vi "SaccadeAnalyser - Main.vi"(8 "error in (no error)":errorcluster, 11 "Data IN":T3={"Impulse Positions"=[{"Start"=5471, "End"=5813, "Impulse Plane"=enum."Yaw", "Impulse Direction +ve?"=FALSE, "Time offset"=0, "Amplitude offset"=0.0}, {"Start"=6974, "End"=7325, "Impulse Plane"=enum."Yaw", "Impulse Direction +ve?"=TRUE, "Time offset"=0, "Amplitude offset"=0.0}, {"Start"=7641, "End"=7980, "Impulse Plane"=enum."Yaw", "Impulse Direction +ve?"=FALSE, "Time offset"=0, "Amplitude offset"=0.0}, {"Start"=9060, "End"=9400, "Impulse Plane"=enum."Yaw", "Impulse Direction +ve?"=FALSE, "Time offset"=0, "Amplitude offset"=0.0}, {"Start"=9938, "End"=10282, "Impulse Plane"=enum."Yaw", "Impulse Direction +ve?"=FALSE, "Time offset"=0, "Amplitude offset"=0.0}, {"Start"=10800, "End"=11142, "Impulse Plane"=enum."Yaw", "Impulse Direction +ve?"=FALSE, "Time offset"=0, "Amplitude offset"=0.0}, {"Start"=11602, "End"=11942, "Impulse Plane"=enum."Yaw", "Impulse Direction +ve?"=TRUE, "Time offset"=0, "Amplitude offset"=0.0}, {"Start"=12449, "End"=12790, "Impulse Plane"=enum."Yaw", "Impulse Direction +ve?"=TRUE, "Time offset"=0, "Amplitude offset"=0.0}, {"Start"=13310, "End"=13653, "Impulse Plane"=enum."Yaw", "Impulse Direction +ve?"=TRUE, "Time offset"=0, "Amplitude offset"=0.0}, {"Start"=14191, "End"=14535, "Impulse Plane"=enum."Yaw", "Impulse Direction +ve?"=TRUE, "Time offset"=0, "Amplitude offset"=0.0}, {"Start"=15040, "End"=15380, "Impulse Plane"=enum."Yaw", "Impulse Direction +ve?"=FALSE, "Time offset"=0, "Amplitude offset"=0.0}, {"Start"=16780, "End"=17124, "Impulse Plane"=enum."Yaw", "Impulse Direction +ve?"=TRUE, "Time offset"=0, "Amplitude offset"=0.0}, {"Start"=17572, "End"=17913, "Impulse Plane"=enum."Yaw", "Impulse Direction +ve?"=FALSE, "Time offset"=0, "Amplitude offset"=0.0}, {"Start"=18369, "End"=18713, "Impulse Plane"=enum."Yaw", "Impulse Direction +ve?"=FALSE, "Time offset"=0, "Amplitude offset"=0.0}, {"Start"=19174, "End"=19519, "Impulse Plane"=enum."Yaw", "Impulse Direction +ve?"=FALSE, "Time offset"=0, "Amplitude offset"=0.0}, {"Start"=19928, "End"=20270, "Impulse Plane"=enum."Yaw", "Impulse Direction +ve?"=TRUE, "Time offset"=0, "Amplitude offset"=0.0}, {"Start"=20762, "End"=21121, "Impulse Plane"=enum."Yaw", "Impulse Direction +ve?"=FALSE, "Time offset"=0, "Amplitude offset"=0.0}, {"Start"=21554, "End"=21888, "Impulse Plane"=enum."Yaw", "Impulse Direction +ve?"=FALSE, "Time offset"=0, "Amplitude offset"=0.0}, {"Start"=22293, "End"=22639, "Impulse Plane"=enum."Yaw", "Impulse Direction +ve?"=TRUE, "Time offset"=0, "Amplitude offset"=0.0}, {"Start"=23109, "End"=23464, "Impulse Plane"=enum."Yaw", "Impulse Direction +ve?"=TRUE, "Time offset"=0, "Amplitude offset"=0.0}, {"Start"=23868, "End"=24215, "Impulse Plane"=enum."Yaw", "Impulse Direction +ve?"=TRUE, "Time offset"=0, "Amplitude offset"=0.0}, {"Start"=24643, "End"=24992, "Impulse Plane"=enum."Yaw", "Impulse Direction +ve?"=FALSE, "Time offset"=0, "Amplitude offset"=0.0}, {"Start"=25685, "End"=26023, "Impulse Plane"=enum."Yaw", "Impulse Direction +ve?"=FALSE, "Time offset"=0, "Amplitude offset"=0.0}, {"Start"=26431, "End"=26768, "Impulse Plane"=enum."Yaw", "Impulse Direction +ve?"=FALSE, "Time offset"=0, "Amplitude offset"=0.0}, {"Start"=27251, "End"=27595, "Impulse Plane"=enum."Yaw", "Impulse Direction +ve?"=FALSE, "Time offset"=0, "Amplitude offset"=0.0}, {"Start"=28832, "End"=29180, "Impulse Plane"=enum."Yaw", "Impulse Direction +ve?"=TRUE, "Time offset"=0, "Amplitude offset"=0.0}, {"Start"=31028, "End"=31383, "Impulse Plane"=enum."LARP", "Impulse Direction +ve?"=FALSE, "Time offset"=0, "Amplitude offset"=0.0}, {"Start"=32603, "End"=32936, "Impulse Plane"=enum."LARP", "Impulse Direction +ve?"=TRUE, "Time offset"=0, "Amplitude offset"=0.0}, {"Start"=33445, "End"=33779, "Impulse Plane"=enum."LARP", "Impulse Direction +ve?"=TRUE, "Time offset"=0, "Amplitude offset"=0.0}, {"Start"=34276, "End"=34629, "Impulse Plane"=enum."LARP", "Impulse Direction +ve?"=FALSE, "Time offset"=0, "Amplitude offset"=0.0}, {"Start"=35114, "End"=35460, "Impulse Plane"=enum."LARP", "Impulse Direction +ve?"=FALSE, "Time offset"=0, "Amplitude offset"=0.0}, {"Start"=35981, "End"=36324, "Impulse Plane"=enum."LARP", "Impulse Direction +ve?"=TRUE, "Time offset"=0, "Amplitude offset"=0.0}, {"Start"=36920, "End"=37249, "Impulse Plane"=enum."LARP", "Impulse Direction +ve?"=TRUE, "Time offset"=0, "Amplitude offset"=0.0}, {"Start"=37988, "End"=38322, "Impulse Plane"=enum."LARP", "Impulse Direction +ve?"=TRUE, "Time offset"=0, "Amplitude offset"=0.0}, {"Start"=38964, "End"=39324, "Impulse Plane"=enum."LARP", "Impulse Direction +ve?"=FALSE, "Time offset"=0, "Amplitude offset"=0.0}, {"Start"=39948, "End"=40284, "Impulse Plane"=enum."LARP", "Impulse Direction +ve?"=TRUE, "Time offset"=0, "Amplitude offset"=0.0}, {"Start"=40958, "End"=41293, "Impulse Plane"=enum."LARP", "Impulse Direction +ve?"=TRUE, "Time offset"=0, "Amplitude offset"=0.0}, {"Start"=41899, "End"=42229, "Impulse Plane"=enum."LARP", "Impulse Direction +ve?"=TRUE, "Time offset"=0, "Amplitude offset"=0.0}, {"Start"=42801, "End"=43154, "Impulse Plane"=enum."LARP", "Impulse Direction +ve?"=FALSE, "Time offset"=0, "Amplitude offset"=0.0}, {"Start"=43641, "End"=43980, "Impulse Plane"=enum."LARP", "Impulse Direction +ve?"=TRUE, "Time offset"=0, "Amplitude offset"=0.0}, {"Start"=44466, "End"=44821, "Impulse Plane"=enum."LARP", "Impulse Direction +ve?"=FALSE, "Time offset"=0, "Amplitude offset"=0.0}, {"Start"=45388, "End"=45722, "Impulse Plane"=enum."LARP", "Impulse Direction +ve?"=TRUE, "Time offset"=0, "Amplitude offset"=0.0}, {"Start"=46149, "End"=46510, "Impulse Plane"=enum."LARP", "Impulse Direction +ve?"=FALSE, "Time offset"=0, "Amplitude offset"=0.0}, {"Start"=47874, "End"=48206, "Impulse Plane"=enum."LARP", "Impulse Direction +ve?"=TRUE, "Time offset"=0, "Amplitude offset"=0.0}, {"Start"=50143, "End"=50479, "Impulse Plane"=enum."RALP", "Impulse Direction +ve?"=TRUE, "Time offset"=0, "Amplitude offset"=0.0}, {"Start"=50976, "End"=51310, "Impulse Plane"=enum."RALP", "Impulse Direction +ve?"=FALSE, "Time offset"=0, "Amplitude offset"=0.0}, {"Start"=51892, "End"=52226, "Impulse Plane"=enum."RALP", "Impulse Direction +ve?"=FALSE, "Time offset"=0, "Amplitude offset"=0.0}, {"Start"=52839, "End"=53171, "Impulse Plane"=enum."RALP", "Impulse Direction +ve?"=FALSE, "Time offset"=0, "Amplitude offset"=0.0}, {"Start"=53676, "End"=54012, "Impulse Plane"=enum."RALP", "Impulse Direction +ve?"=TRUE, "Time offset"=0, "Amplitude offset"=0.0}, {"Start"=54530, "End"=54877, "Impulse Plane"=enum."RALP", "Impulse Direction +ve?"=FALSE, "Time offset"=0, "Amplitude offset"=0.0}, {"Start"=55371, "End"=55711, "Impulse Plane"=enum."RALP", "Impulse Direction +ve?"=TRUE, "Time offset"=0, "Amplitude offset"=0.0}, {"Start"=56153, "End"=56482, "Impulse Plane"=enum."RALP", "Impulse Direction +ve?"=FALSE, "Time offset"=0, "Amplitude offset"=0.0}, {"Start"=57053, "End"=57390, "Impulse Plane"=enum."RALP", "Impulse Direction +ve?"=FALSE, "Time offset"=0, "Amplitude offset"=0.0}, {"Start"=57954, "End"=58292, "Impulse Plane"=enum."RALP", "Impulse Direction +ve?"=FALSE, "Time offset"=0, "Amplitude offset"=0.0}, {"Start"=58794, "End"=59130, "Impulse Plane"=enum."RALP", "Impulse Direction +ve?"=TRUE, "Time offset"=0, "Amplitude offset"=0.0}, {"Start"=59587, "End"=59931, "Impulse Plane"=enum."RALP", "Impulse Direction +ve?"=TRUE, "Time offset"=0, "Amplitude offset"=0.0}, {"Start"=60399, "End"=60744, "Impulse Plane"=enum."RALP", "Impulse Direction +ve?"=FALSE, "Time offset"=0, "Amplitude offset"=0.0}, {"Start"=61218, "End"=61559, "Impulse Plane"=enum."RALP", "Impulse Direction +ve?"=FALSE, "Time offset"=0, "Amplitude offset"=0.0}, {"Start"=62100, "End"=62442, "Impulse Plane"=enum."RALP", "Impulse Direction +ve?"=FALSE, "Time offset"=0, "Amplitude offset"=0.0}, {"Start"=62989, "End"=63322, "Impulse Plane"=enum."RALP", "Impulse Direction +ve?"=FALSE, "Time offset"=0, "Amplitude offset"=0.0}, {"Start"=63787, "End"=64136, "Impulse Plane"=enum."RALP", "Impulse Direction +ve?"=TRUE, "Time offset"=0, "Amplitude offset"=0.0}, {"Start"=64603, "End"=64953, "Impulse Plane"=enum."RALP", "Impulse Direction +ve?"=FALSE, "Time offset"=0, "Amplitude offset"=0.0}, {"Start"=65462, "End"=65795, "Impulse Plane"=enum."RALP", "Impulse Direction +ve?"=FALSE, "Time offset"=0, "Amplitude offset"=0.0}, {"Start"=66308, "End"=66645, "Impulse Plane"=enum."RALP", "Impulse Direction +ve?"=FALSE, "Time offset"=0, "Amplitude offset"=0.0}, {"Start"=67052, "End"=67402, "Impulse Plane"=enum."RALP", "Impulse Direction +ve?"=TRUE, "Time offset"=0, "Amplitude offset"=0.0}], "No. Imp"=15, "Parameter Time Series"=[{"time offset"=0.0, "Offset"=0.0, "Gain"=1.0, "inverse"=FALSE, "filter data"=FALSE, "dots"=FALSE, "interpolate"=FALSE, "List 1"=5, "Color Box"=6618880, "Boolean"=TRUE}, {"time offset"=0.0, "Offset"=0.0, "Gain"=1.0, "inverse"=FALSE, "filter data"=FALSE, "dots"=FALSE, "interpolate"=FALSE, "List 1"=6, "Color Box"=6618880, "Boolean"=FALSE}, {"time offset"=0.0, "Offset"=0.0, "Gain"=1.0, "inverse"=FALSE, "filter data"=FALSE, "dots"=FALSE, "interpolate"=FALSE, "List 1"=7, "Color Box"=6618880, "Boolean"=FALSE}, {"time offset"=0.0, "Offset"=0.0, "Gain"=1.0, "inverse"=FALSE, "filter data"=FALSE, "dots"=FALSE, "interpolate"=FALSE, "List 1"=13, "Color Box"=16777224, "Boolean"=TRUE}, {"time offset"=0.0, "Offset"=0.0, "Gain"=1.0, "inverse"=FALSE, "filter data"=FALSE, "dots"=FALSE, "interpolate"=FALSE, "List 1"=14, "Color Box"=16777224, "Boolean"=FALSE}, {"time offset"=0.0, "Offset"=0.0, "Gain"=1.0, "inverse"=FALSE, "filter data"=FALSE, "dots"=FALSE, "interpolate"=FALSE, "List 1"=15, "Color Box"=16777224, "Boolean"=FALSE}], "Parameter Impuls Series"=[{"Color"=6618880, "Visible"=TRUE, "Channel"=1, "Invert"=FALSE, "Desaccade"=FALSE, "Offset"=0.0, "Gain"=1.0}, {"Color"=6618880, "Visible"=FALSE, "Channel"=6, "Invert"=FALSE, "Desaccade"=FALSE, "Offset"=0.0, "Gain"=1.0}, {"Color"=6618880, "Visible"=FALSE, "Channel"=7, "Invert"=FALSE, "Desaccade"=FALSE, "Offset"=0.0, "Gain"=1.0}, {"Color"=16777224, "Visible"=TRUE, "Channel"=13, "Invert"=FALSE, "Desaccade"=FALSE, "Offset"=0.0, "Gain"=1.0}, {"Color"=16777224, "Visible"=FALSE, "Channel"=14, "Invert"=FALSE, "Desaccade"=FALSE, "Offset"=0.0, "Gain"=1.0}, {"Color"=16777224, "Visible"=FALSE, "Channel"=15, "Invert"=FALSE, "Desaccade"=FALSE, "Offset"=0.0, "Gain"=1.0}], "Experiment Parameters"={"Freq"=0.0, "Vel"=0, "Acc"=0, "Stimulus"="Head Impulse"}, "Autosort File"=refnum, "Data File"={"Data Channels"=array34x71049[2415666 elements], "Sample Rate"=500, "Channel List"=["Hz Position-in-Head", "Hz Velocity-in-Head", "Hy Position-in-Head", "Hy Velocity-in-Head", "Hx Position-in-Head", "Hx Velocity-in-Head", "Hl Velocity-in-Head", "Hr Velocity-in-Head", "Lx Position-in-Head", "Ly Position-in-Head", "Lz Position-in-Head", "Lx Velocity-in-Head", "Ly Velocity-in-Head", "Lz Velocity-in-Head", "Ll Velocity-in-Head", "Lr Velocity-in-Head", "Rx Position-in-Head", "Ry Position-in-Head", "Rz Position-in-Head", "Rx Velocity-in-Head", "Ry Velocity-in-Head", "Rz Velocity-in-Head", "Rl Velocity-in-Head", "Rr Velocity-in-Head", "Target on/off", "aux input 1", "aux input 2", " ", "", "", "", "Target Hor", "Target Ver", ""]}, "Experiment data path"=path "C:/Users/w.figtree/Desktop/Coils Data/3", "Image data path"=path "/Macintosh HD/Users/patrick/Studium/Diploma Thesis/Data Analysis", "LVS data path"=path "/Macintosh HD/Users/patrick/Studium/Diploma Thesis/Data Analysis", "Raw copy path"=path "/Macintosh HD/Users/patrick/Studium/Diploma Thesis/Data Analysis", "filename"="passive_lvs.lvs", "desaccading parameters"={"Tolerance"=3, "Acc Range"=7000.0, "Sample Rate"=500, "Impulse Plane 2"=enum."Yaw", "Impulse dir"=FALSE}, "Experiment Parameters 2"={"Subject"="SE Trial Short Term", "Strain"="", "Rotation plane"="", "Experimenter"=" ", "Trial"=0.0, "Time"=0.0}, "Excel"={"Excel._Application"=refnum, "Use Excel"=TRUE, "Worksheet SINE"=refnum, "Row SINE"=0, "Worksheet TRANS"=refnum, "Row TRANS"=0}, "Session Config File"=refnum, "Autosort Parameter Set"=4, "EMA Version"="EMA 2016a", "desacc "={"Threshold 1 [Acc]"=7000.0, "Threshold 2 [% of TH1]"=60, "tolerance"=3, "Search WD "=0.1, " always use TH2"=FALSE, "Range"=3.0, "Max time"=120.0, "Min time"=20.0, "Velocity Threshold"=150}, "Cycle Nr for Saccades"={"POS"=0, "NEG"=0}, "calibration name"="u_calibration_1_p00001s001_calib.mat", "Excel"=refnum} {"Parameter Time Series"."time offset" format="%.3f"; "Parameter Time Series"."Gain" format="%.1f"; "Parameter Time Series"."Offset" format="%.1f"; "Parameter Time Series"."List 1" items=["Motor-Pos", "Motor-Vel", "Lx Position-in-Head", "Ly Position-in-Head", "Lz Position-in-Head", "Lx Velocity-in-Head", "Ly Velocity-in-Head", "Lz Velocity-in-Head", "Ll Velocity-in-Head", "Lr Velocity-in-Head", "Lx Accel-in-Head", "Ly Accel-in-Head", "Lz Accel-in-Head", "Rx Position-in-Head", "Ry Position-in-Head", "Rz Position-in-Head", "Rx Velocity-in-Head", "Ry Velocity-in-Head", "Rz Velocity-in-Head", "Rl Velocity-in-Head", "Rr Velocity-in-Head", "Rx Accel-in-Head", "Ry Accel-in-Head", "Rz Accel-in-Head", "Global Trigger", "", "", ""]; "Parameter Impuls Series"."Gain" format="%.1f"; "Parameter Impuls Series"."Offset" format="%.1f"}) -> (0 "error out":errorcluster, 3 "Data OUT":T3={"Impulse Positions"=[{"Start"=5471, "End"=5813, "Impulse Plane"=enum."Yaw", "Impulse Direction +ve?"=FALSE, "Time offset"=0, "Amplitude offset"=0.0}, {"Start"=6974, "End"=7325, "Impulse Plane"=enum."Yaw", "Impulse Direction +ve?"=TRUE, "Time offset"=0, "Amplitude offset"=0.0}, {"Start"=7641, "End"=7980, "Impulse Plane"=enum."Yaw", "Impulse Direction +ve?"=FALSE, "Time offset"=0, "Amplitude offset"=0.0}, {"Start"=9060, "End"=9400, "Impulse Plane"=enum."Yaw", "Impulse Direction +ve?"=FALSE, "Time offset"=0, "Amplitude offset"=0.0}, {"Start"=9938, "End"=10282, "Impulse Plane"=enum."Yaw", "Impulse Direction +ve?"=FALSE, "Time offset"=0, "Amplitude offset"=0.0}, {"Start"=10800, "End"=11142, "Impulse Plane"=enum."Yaw", "Impulse Direction +ve?"=FALSE, "Time offset"=0, "Amplitude offset"=0.0}, {"Start"=11602, "End"=11942, "Impulse Plane"=enum."Yaw", "Impulse Direction +ve?"=TRUE, "Time offset"=0, "Amplitude offset"=0.0}, {"Start"=12449, "End"=12790, "Impulse Plane"=enum."Yaw", "Impulse Direction +ve?"=TRUE, "Time offset"=0, "Amplitude offset"=0.0}, {"Start"=13310, "End"=13653, "Impulse Plane"=enum."Yaw", "Impulse Direction +ve?"=TRUE, "Time offset"=0, "Amplitude offset"=0.0}, {"Start"=14191, "End"=14535, "Impulse Plane"=enum."Yaw", "Impulse Direction +ve?"=TRUE, "Time offset"=0, "Amplitude offset"=0.0}, {"Start"=15040, "End"=15380, "Impulse Plane"=enum."Yaw", "Impulse Direction +ve?"=FALSE, "Time offset"=0, "Amplitude offset"=0.0}, {"Start"=16780, "End"=17124, "Impulse Plane"=enum."Yaw", "Impulse Direction +ve?"=TRUE, "Time offset"=0, "Amplitude offset"=0.0}, {"Start"=17572, "End"=17913, "Impulse Plane"=enum."Yaw", "Impulse Direction +ve?"=FALSE, "Time offset"=0, "Amplitude offset"=0.0}, {"Start"=18369, "End"=18713, "Impulse Plane"=enum."Yaw", "Impulse Direction +ve?"=FALSE, "Time offset"=0, "Amplitude offset"=0.0}, {"Start"=19174, "End"=19519, "Impulse Plane"=enum."Yaw", "Impulse Direction +ve?"=FALSE, "Time offset"=0, "Amplitude offset"=0.0}, {"Start"=19928, "End"=20270, "Impulse Plane"=enum."Yaw", "Impulse Direction +ve?"=TRUE, "Time offset"=0, "Amplitude offset"=0.0}, {"Start"=20762, "End"=21121, "Impulse Plane"=enum."Yaw", "Impulse Direction +ve?"=FALSE, "Time offset"=0, "Amplitude offset"=0.0}, {"Start"=21554, "End"=21888, "Impulse Plane"=enum."Yaw", "Impulse Direction +ve?"=FALSE, "Time offset"=0, "Amplitude offset"=0.0}, {"Start"=22293, "End"=22639, "Impulse Plane"=enum."Yaw", "Impulse Direction +ve?"=TRUE, "Time offset"=0, "Amplitude offset"=0.0}, {"Start"=23109, "End"=23464, "Impulse Plane"=enum."Yaw", "Impulse Direction +ve?"=TRUE, "Time offset"=0, "Amplitude offset"=0.0}, {"Start"=23868, "End"=24215, "Impulse Plane"=enum."Yaw", "Impulse Direction +ve?"=TRUE, "Time offset"=0, "Amplitude offset"=0.0}, {"Start"=24643, "End"=24992, "Impulse Plane"=enum."Yaw", "Impulse Direction +ve?"=FALSE, "Time offset"=0, "Amplitude offset"=0.0}, {"Start"=25685, "End"=26023, "Impulse Plane"=enum."Yaw", "Impulse Direction +ve?"=FALSE, "Time offset"=0, "Amplitude offset"=0.0}, {"Start"=26431, "End"=26768, "Impulse Plane"=enum."Yaw", "Impulse Direction +ve?"=FALSE, "Time offset"=0, "Amplitude offset"=0.0}, {"Start"=27251, "End"=27595, "Impulse Plane"=enum."Yaw", "Impulse Direction +ve?"=FALSE, "Time offset"=0, "Amplitude offset"=0.0}, {"Start"=28832, "End"=29180, "Impulse Plane"=enum."Yaw", "Impulse Direction +ve?"=TRUE, "Time offset"=0, "Amplitude offset"=0.0}, {"Start"=31028, "End"=31383, "Impulse Plane"=enum."LARP", "Impulse Direction +ve?"=FALSE, "Time offset"=0, "Amplitude offset"=0.0}, {"Start"=32603, "End"=32936, "Impulse Plane"=enum."LARP", "Impulse Direction +ve?"=TRUE, "Time offset"=0, "Amplitude offset"=0.0}, {"Start"=33445, "End"=33779, "Impulse Plane"=enum."LARP", "Impulse Direction +ve?"=TRUE, "Time offset"=0, "Amplitude offset"=0.0}, {"Start"=34276, "End"=34629, "Impulse Plane"=enum."LARP", "Impulse Direction +ve?"=FALSE, "Time offset"=0, "Amplitude offset"=0.0}, {"Start"=35114, "End"=35460, "Impulse Plane"=enum."LARP", "Impulse Direction +ve?"=FALSE, "Time offset"=0, "Amplitude offset"=0.0}, {"Start"=35981, "End"=36324, "Impulse Plane"=enum."LARP", "Impulse Direction +ve?"=TRUE, "Time offset"=0, "Amplitude offset"=0.0}, {"Start"=36920, "End"=37249, "Impulse Plane"=enum."LARP", "Impulse Direction +ve?"=TRUE, "Time offset"=0, "Amplitude offset"=0.0}, {"Start"=37988, "End"=38322, "Impulse Plane"=enum."LARP", "Impulse Direction +ve?"=TRUE, "Time offset"=0, "Amplitude offset"=0.0}, {"Start"=38964, "End"=39324, "Impulse Plane"=enum."LARP", "Impulse Direction +ve?"=FALSE, "Time offset"=0, "Amplitude offset"=0.0}, {"Start"=39948, "End"=40284, "Impulse Plane"=enum."LARP", "Impulse Direction +ve?"=TRUE, "Time offset"=0, "Amplitude offset"=0.0}, {"Start"=40958, "End"=41293, "Impulse Plane"=enum."LARP", "Impulse Direction +ve?"=TRUE, "Time offset"=0, "Amplitude offset"=0.0}, {"Start"=41899, "End"=42229, "Impulse Plane"=enum."LARP", "Impulse Direction +ve?"=TRUE, "Time offset"=0, "Amplitude offset"=0.0}, {"Start"=42801, "End"=43154, "Impulse Plane"=enum."LARP", "Impulse Direction +ve?"=FALSE, "Time offset"=0, "Amplitude offset"=0.0}, {"Start"=43641, "End"=43980, "Impulse Plane"=enum."LARP", "Impulse Direction +ve?"=TRUE, "Time offset"=0, "Amplitude offset"=0.0}, {"Start"=44466, "End"=44821, "Impulse Plane"=enum."LARP", "Impulse Direction +ve?"=FALSE, "Time offset"=0, "Amplitude offset"=0.0}, {"Start"=45388, "End"=45722, "Impulse Plane"=enum."LARP", "Impulse Direction +ve?"=TRUE, "Time offset"=0, "Amplitude offset"=0.0}, {"Start"=46149, "End"=46510, "Impulse Plane"=enum."LARP", "Impulse Direction +ve?"=FALSE, "Time offset"=0, "Amplitude offset"=0.0}, {"Start"=47874, "End"=48206, "Impulse Plane"=enum."LARP", "Impulse Direction +ve?"=TRUE, "Time offset"=0, "Amplitude offset"=0.0}, {"Start"=50143, "End"=50479, "Impulse Plane"=enum."RALP", "Impulse Direction +ve?"=TRUE, "Time offset"=0, "Amplitude offset"=0.0}, {"Start"=50976, "End"=51310, "Impulse Plane"=enum."RALP", "Impulse Direction +ve?"=FALSE, "Time offset"=0, "Amplitude offset"=0.0}, {"Start"=51892, "End"=52226, "Impulse Plane"=enum."RALP", "Impulse Direction +ve?"=FALSE, "Time offset"=0, "Amplitude offset"=0.0}, {"Start"=52839, "End"=53171, "Impulse Plane"=enum."RALP", "Impulse Direction +ve?"=FALSE, "Time offset"=0, "Amplitude offset"=0.0}, {"Start"=53676, "End"=54012, "Impulse Plane"=enum."RALP", "Impulse Direction +ve?"=TRUE, "Time offset"=0, "Amplitude offset"=0.0}, {"Start"=54530, "End"=54877, "Impulse Plane"=enum."RALP", "Impulse Direction +ve?"=FALSE, "Time offset"=0, "Amplitude offset"=0.0}, {"Start"=55371, "End"=55711, "Impulse Plane"=enum."RALP", "Impulse Direction +ve?"=TRUE, "Time offset"=0, "Amplitude offset"=0.0}, {"Start" (continued)
        n226 = case shown="False" w362 {
          tunnel: [w373 w391] -> w357
          tunnel: w363 -> [w370 _]
          frame False {
            # "Iterate by stat rather than saccade"
            # "Saccades included -> Analyse them."
            n227 = local read "enum_summaryType"() -> (w372:enum16{"Mean", "Median"})
            n228 = Transpose 2D Array(2D array=w370) -> (transposed array=w371:dbl[][])
            n229 = for {
              tunnel: w371 -> [w377] mode=indexing
              tunnel: w372 -> [w379]
              tunnel: [w378] -> w373 mode=indexing
              # "For each stat -> Calculate the summary"
              n230 = for {
                tunnel: w377 -> [w390] mode=indexing
                tunnel: [w390] -> w375 mode=indexing if=w388
                # "Filter out NaNs"
                n231 = Not A Number/Path/Refnum?(number/path/refnum=w390) -> (NaN/Path/Refnum?=w389:bool)
                n232 = Not(x=w389) -> (.not. x?=w388:bool)
              }
              n233 = Array Size(array=w375) -> (size(s)=w376:i32)
              n234 = Equal To 0?(x=w376) -> (x = 0?=w374:bool)
              n235 = case shown="False" w374 {
                tunnel: w379 -> [w382 _]
                tunnel: [w381 nan ("median")] -> w378
                tunnel: w375 -> [w380 _]
                frame False {
                  # "Do analysis"
                  n236 = case shown="\"Mean\", Default" w382 {
                    tunnel: w380 -> [w383 w386]
                    tunnel: [w384 w385] -> w381
                    frame "Mean", Default {
                      n237 = call-poly <vilib>:"Mean.vi"("X"=w383) -> ("mean"=w384:dbl)  [unwired: 1 out]
                    }
                    frame "Median" {
                      n238 = call <vilib>:"Median.vi"("X"=w386) -> ("median"=w385:dbl)  [unwired: 1 out]
                    }
                  }
                }
                frame True {
                  # "No data -> NaN"
                }
              }
            }
          }
          frame True {
            # "No saccades -> Output NaN."
            n239 = Initialize Array(nan, 5 ("dimension size")) -> (w391:dbl[])
          }
        }
        n240 = Index Array(array=w357) -> (element #1=w356:dbl, element #2=w355:dbl, element #3=w354:dbl, element #4=w353:dbl, element #5=w352:dbl)  [unwired: 5 in]
        n241 = Bundle By Name(cluster=w367, "Summary.Num Impulses"=w359, "Summary.Num Saccades"=w358, "Summary.Onset (ms)"=w356, "Summary.Duration (ms)"=w355, "Summary.Vel (°/s)"=w354, "Summary.Amplitude (°)"=w353, "Summary.Gain"=w352) -> (w366:T6)
      }
      frame "Calc Saccade Group Stats" {
        # "Calculates the summary statistics across all the saccades grouped by sequence number."
        n242 = Unbundle By Name(w405) -> ("Saccades"=w407:T8[])
        n243 = local read "num_groups"() -> (w406:u32)
        n244 = for {
          N: w406 -> [_]
          tunnel: w407 -> [w419]
          tunnel: [w410] -> w403 mode=indexing
          i -> [w418]
          (unwired) T9 {"Num Impulses"=0.0, "Num Saccades"=0.0, "Onset (ms)"=0.0, "Onset SD (ms)"=0.0, "Duration (ms)"=0.0, "Duration SD (ms)"=0.0, "Vel (°/s)"=0.0, "Vel SD (°/s)"=0.0, "Amplitude (°)"=0.0, "Amplitude SD (°)"=0.0, "Gain"=0.0, "Gain SD"=0.0} ("Summary")
          # "For each group, calculate stats..."
          n245 = for {
            tunnel: w419 -> [w453] mode=indexing
            tunnel: w418 -> [w461]
            tunnel: [w452] -> w415 mode=indexing if=w450
            tunnel: [w451] -> w416 mode=indexing if=w450
            # "Saccade must be included and match the group number"
            # "Get data from saccades in sequence groups"
            n246 = Unbundle By Name(w453) -> ("Impulse"=w451:i32, "Onset (ms)"=w458:dbl, "Duration (ms)"=w457:dbl, "Vel (°/s)"=w456:dbl, "Amplitude (°)"=w455:dbl, "Gain"=w454:dbl)
            n247 = Unbundle By Name(w453) -> ("Included?"=w460:bool, "Sequence #"=w462:dbl)
            n248 = Equal?(x=w462, y=w461) -> (x = y?=w459:bool)
            n249 = Compound Arithmetic op=AND(w460, w459) -> (w450:bool)
            n250 = Build Array(w458, w457, w456, w455, w454) -> (w452:dbl[])
          }
          n251 = call-poly <userlib>:"Remove Duplicates from 1D Array__ogtk.vi"("Input Array"=w416) -> ("Output Array"=w417:i32[])  [unwired: 1 out]
          n252 = Array Size(array=w417) -> (size(s)=w413:i32)
          n253 = Array Size(array=w416) -> (size(s)=w412:i32)
          n254 = case shown="Default" w412 {
            tunnel: [w420 w447] -> w414
            tunnel: w415 -> [w423 _]
            frame Default {
              # "Iterate by stat rather than saccade"
              # "Saccades included -> Analyse them."
              n255 = local read "enum_summaryType"() -> (w425:enum16{"Mean", "Median"})
              n256 = Transpose 2D Array(2D array=w423) -> (transposed array=w424:dbl[][])
              n257 = for {
                tunnel: w424 -> [w430] mode=indexing
                tunnel: w425 -> [w432]
                tunnel: [w431] -> w422 mode=indexing
                tunnel: [w426] -> w421 mode=indexing
                # "For each stat -> Calculate the summary"
                n258 = for {
                  tunnel: w430 -> [w446] mode=indexing
                  tunnel: [w446] -> w428 mode=indexing if=w444
                  # "Filter out NaNs"
                  n259 = Not A Number/Path/Refnum?(number/path/refnum=w446) -> (NaN/Path/Refnum?=w445:bool)
                  n260 = Not(x=w445) -> (.not. x?=w444:bool)
                }
                n261 = Array Size(array=w428) -> (size(s)=w429:i32)
                n262 = Equal To 0?(x=w429) -> (x = 0?=w427:bool)
                n263 = case shown="False" w427 {
                  tunnel: w432 -> [w436 _]
                  tunnel: [w435 w443] -> w431
                  tunnel: w428 -> [w434 _]
                  tunnel: [w433 w443] -> w426
                  frame False {
                    # "Do analysis"
                    n264 = case shown="\"Median\"" w436 {
                      tunnel: w434 -> [w438 w441]
                      tunnel: [w439 w442] -> w435
                      tunnel: [w437 w440] -> w433
                      frame "Mean", Default {
                        n265 = call <vilib>:"Std Deviation and Variance.vi"("X"=w438) -> ("mean"=w439:dbl, "standard deviation"=w437:dbl)  [unwired: 1 in, 1 out]
                      }
                      frame "Median" {
                        n266 = call <vilib>:"Median.vi"("X"=w441) -> ("median"=w442:dbl)  [unwired: 1 out]
                        n267 = call <vilib>:"Std Deviation and Variance.vi"("X"=w441) -> ("standard deviation"=w440:dbl)  [unwired: 1 in, 2 out]
                      }
                    }
                  }
                  frame True {
                    w443 = nan ("median")
                    # "No data -> NaN"
                  }
                }
              }
              n268 = Interleave 1D Arrays(w422, w421) -> (w420:dbl[])
            }
            frame 0 {
              # "No saccades -> Output NaN."
              n269 = Initialize Array(nan, 10 ("dimension size")) -> (w447:dbl[])
            }
          }
          n270 = Build Array (concatenate)(w413, w412, w414) -> (w411:dbl[])
          n271 = Array To Cluster(array=w411) -> (cluster=w410:T22)
        }
        n272 = Bundle By Name(cluster=w405, "Group Summary"=w403) -> (w404:T6)
      }
      frame "DO - Draw" {
        w463 = T10[] [enum."Halt Panel Updates", enum."Disable Controls", enum."Clear Plot", enum."Plot Selected Saccade", enum."Plot Selected Saccade Siblings", enum."Plot Saccade Data", enum."Plot Impulse Data", enum."Fill Saccade MCLB", enum."Fill Summary Stats", enum."Enable Controls", enum."Give MCLB Focus", enum."Resume Panel Updates"] items=["Initialise", "Quit", "DO - Analysis", "DO - Summary Analysis", "Load Channel Data", "Find Impulses", "Find Saccades", "Sequence Saccades", "Calc Saccade Summary Stats", "Calc Saccade Group Stats", "DO - Draw", "Clear Plot", "Plot Selected Saccade", "Plot Selected Saccade Siblings", "Plot Impulse Data", "Plot Saccade Data", "Fill Saccade MCLB", "Fill Summary Stats", "Give MCLB Focus", "Halt Panel Updates", "Resume Panel Updates", "Disable Controls", "Enable Controls", "Toggle Saccade", "DO - Export Summary", "Export - Open Summary", "Export - Summary", "DO - Export Saccades", "Export - Open Saccades", "Export - Saccades", "DO - Export Group", "Export - Open Group", "Export - Group", "Do - Export All"] ("element")
        # "Enqueue draw process states."
        n273 = for {
          tunnel: w464 -> [w469]
          tunnel: w463 -> [w468] mode=indexing
          n274 = Enqueue Element(queue=w469, element=w468) -> ()  [unwired: 2 in, 3 out]
        }
      }
      frame "Clear Plot" {
        # "Clears all data from the XY graph."
        n275 = local write "graph"(cluster{dbl[], dbl[]}[] [] ("graph")) -> ()
      }
      frame "Plot Selected Saccade" {
        # "Check selected value is in range"
        # "Plot (with emphasis) the saccade selected in the MCLB."
        n276 = Unbundle By Name(w481) -> ("Sample Rate (Hz)"=w485:dbl, "Saccades"=w478:T8[], "Impulse Data"=w484:refnum<data-value>, "Palette.Selected Saccade"=w483:u32, "Palette.Excluded Saccade"=w482:u32)
        n277 = local read "mclb_saccades"() -> (w480:i32)
        n278 = Array Size(array=w478) -> (size(s)=w477:i32)
        n279 = Decrement(x=w477) -> (x-1=w476:i32)
        n280 = In Range and Coerce(upper limit=w476, x=w480, lower limit=0) -> (coerced(x)=w475:i32, In Range?=w474:bool)
        n281 = case shown="True" w474 {
          tunnel: w485 -> [_ w507]
          tunnel: w484 -> [_ w506]
          tunnel: w478 -> [_ w491]
          tunnel: w483 -> [_ w504]
          tunnel: w482 -> [_ w503]
          tunnel: w475 -> [_ w490]
          frame False {
          }
          frame True {
            # "emphasis thickness"
            n282 = Index Array(array=w491, index=w490) -> (element=w489:T8)
            n283 = Unbundle By Name(w489) -> ("Included?"=w493:bool)
            n284 = Select(t=w504, s=w493, f=w503) -> (s? t:f=w492:u32)
            n285 = Bundle By Name(cluster=T17 {"Plot.Anti-aliased"=FALSE, "Plot.Bar Plot Style"=0, "Plot.Digital Line Style"=0, "Plot.Digital Transition Location"=0, "Plot.Digital Transition Type"=0, "Plot.Fill To"=-1, "Plot.Fill/Point Color"=0, "Plot.Label Format"=0, "Plot.Line Style"=0, "Plot.Line Width"=0, "Plot.Plot Color"=0, "Plot.Plot Interpolation"=2, "Plot.Plot Name"="", "Plot.Point Style"=0, "Plot.Visible"=TRUE} ("Style"), "Plot.Plot Color"=w492, "Plot.Line Width"=u8 4) -> (w494:T17)
            n286 = Unbundle By Name(w489) -> ("Start (idx)"=w502:dbl, "End (idx)"=w501:dbl)
            n287 = call "ImpulseData - Get Saccade Trace.vi"("Saccade in"=w489, "Impulse Data"=w506) -> ("Response Data"=w497:dbl[])  [unwired: 4 in, 4 out]
            n288 = call "Build dt Ramp.vi"("Stop idx"=w501, "Start idx (0)"=w502, "Frequency (Hz)"=w507) -> ("Ramp (s)"=w499:dbl[])  [unwired: 7 in, 1 out]
            n289 = Multiply(x=w499, y=1000.0) -> (x*y=w500:dbl[])
            n290 = control-ref of="graph"() -> (w505:refnum<vi>)
            n291 = Bundle(w500, "Response Data"=w497) -> (w496:cluster{dbl[], "Response Data":dbl[]})  [unwired: 1 in]
            n292 = call "XY Graph - Append Plot.vi"("Style"=w494, "Data"=w496, "XYGraph Refnum in"=w505) -> ()  [unwired: 7 in, 2 out]
          }
        }
      }
      frame "Plot Selected Saccade Siblings" {
        # "Check selected value is in range"
        # "Plot any saccades occuring in the same impulse as the saccade selected in the MCLB."
        n293 = Unbundle By Name(w508) -> ("Sample Rate (Hz)"=w519:dbl, "Saccades"=w513:T8[], "Impulse Data"=w518:refnum<data-value>, "Palette.Sibling Saccade"=w517:u32, "Palette.Excluded Saccade"=w516:u32)
        n294 = local read "mclb_saccades"() -> (w515:i32)
        n295 = Array Size(array=w513) -> (size(s)=w512:i32)
        n296 = Decrement(x=w512) -> (x-1=w511:i32)
        n297 = In Range and Coerce(upper limit=w511, x=w515, lower limit=0) -> (coerced(x)=w510:i32, In Range?=w509:bool)
        n298 = case shown="True" w509 {
          tunnel: w519 -> [_ w529]
          tunnel: w518 -> [_ w528]
          tunnel: w513 -> [_ w525]
          tunnel: w517 -> [_ w527]
          tunnel: w516 -> [_ w526]
          tunnel: w510 -> [_ w524]
          frame False {
          }
          frame True {
            n299 = Delete From Array(array=w525, index=w524) -> (deleted portion=w523:T8, array with subset deleted=w522:T8[])  [unwired: 1 in]
            n300 = for {
              tunnel: w529 -> [w538]
              tunnel: w528 -> [w537]
              tunnel: w527 -> [w536]
              tunnel: w526 -> [w535]
              tunnel: w522 -> [w533] mode=indexing
              tunnel: w523 -> [w534]
              n301 = Unbundle By Name(w534) -> ("Impulse"=w532:i32)
              n302 = Unbundle By Name(w533) -> ("Impulse"=w531:i32)
              n303 = Equal?(x=w532, y=w531) -> (x = y?=w530:bool)
              n304 = case shown="True" w530 {
                tunnel: w538 -> [_ w557]
                tunnel: w537 -> [_ w556]
                tunnel: w536 -> [_ w554]
                tunnel: w535 -> [_ w553]
                tunnel: w533 -> [_ w541]
                frame False {
                }
                frame True {
                  # "Markers only, Filled markers"
                  n305 = Unbundle By Name(w541) -> ("Start (idx)"=w552:dbl, "End (idx)"=w551:dbl)
                  n306 = call "ImpulseData - Get Saccade Trace.vi"("Saccade in"=w541, "Impulse Data"=w556) -> ("Response Data"=w547:dbl[])  [unwired: 4 in, 4 out]
                  n307 = Unbundle By Name(w541) -> ("Included?"=w543:bool)
                  n308 = Select(t=w554, s=w543, f=w553) -> (s? t:f=w542:u32)
                  n309 = call "Build dt Ramp.vi"("Stop idx"=w551, "Start idx (0)"=w552, "Frequency (Hz)"=w557) -> ("Ramp (s)"=w549:dbl[])  [unwired: 7 in, 1 out]
                  n310 = Bundle By Name(cluster=T17 {"Plot.Anti-aliased"=FALSE, "Plot.Bar Plot Style"=0, "Plot.Digital Line Style"=0, "Plot.Digital Transition Location"=0, "Plot.Digital Transition Type"=0, "Plot.Fill To"=-1, "Plot.Fill/Point Color"=0, "Plot.Label Format"=0, "Plot.Line Style"=0, "Plot.Line Width"=0, "Plot.Plot Color"=0, "Plot.Plot Interpolation"=2, "Plot.Plot Name"="", "Plot.Point Style"=0, "Plot.Visible"=TRUE} ("Style"), "Plot.Fill/Point Color"=w542, "Plot.Plot Interpolation"=u8 0 ("Plot.Line Style"), "Plot.Point Style"=u8 2) -> (w544:T17)
                  n311 = Multiply(x=w549, y=1000.0) -> (x*y=w550:dbl[])
                  n312 = Bundle(w550, "Response Data"=w547) -> (w546:cluster{dbl[], "Response Data":dbl[]})  [unwired: 1 in]
                  n313 = control-ref of="graph"() -> (w555:refnum<vi>)
                  n314 = call "XY Graph - Append Plot.vi"("Style"=w544, "Data"=w546, "XYGraph Refnum in"=w555) -> ()  [unwired: 7 in, 2 out]
                }
              }
            }
          }
        }
      }
      frame "Plot Impulse Data" {
        w562 = T17 {"Plot.Anti-aliased"=FALSE, "Plot.Bar Plot Style"=0, "Plot.Digital Line Style"=0, "Plot.Digital Transition Location"=0, "Plot.Digital Transition Type"=0, "Plot.Fill To"=-1, "Plot.Fill/Point Color"=0, "Plot.Label Format"=0, "Plot.Line Style"=0, "Plot.Line Width"=0, "Plot.Plot Color"=0, "Plot.Plot Interpolation"=2, "Plot.Plot Name"="", "Plot.Point Style"=0, "Plot.Visible"=TRUE} ("Style")
        # "Build time point array"
        # "Plot impulse data to the graph."
        n315 = Unbundle By Name(w570) -> ("Impulse Data"=w569:refnum<data-value>, "Sample Rate (Hz)"=w564:dbl, "Impulse Duration (samples)"=w568:i32, "Palette.Response"=w561:u32, "Palette.Stimulus"=w560:u32)
        n316 = Bundle By Name(cluster=w562, "Plot.Plot Color"=w561) -> (w559:T17)
        n317 = Bundle By Name(cluster=w562, "Plot.Plot Color"=w560) -> (w558:T17)
        n318 = call "Build dt Ramp.vi"("Stop idx"=w568, "Frequency (Hz)"=w564) -> ("Ramp (s)"=w567:dbl[])  [unwired: 8 in, 1 out]
        n319 = Multiply(x=1000.0, y=w567) -> (x*y=w565:dbl[])
        n320 = control-ref of="graph"() -> (w563:refnum<vi>)
        n321 = in-place {
          in-place-border: w565 -> [w576]
          in-place-border: w563 -> [w575]
          in-place-border: w559 -> [w574]
          in-place-border: w558 -> [w573]
          n322 = in-place-dvr #5(w569) -> (w578:T15[])  [unwired: 1 out]
          n323 = for {
            tunnel: w578 -> [w587] mode=indexing
            tunnel: [w587] -> w577 mode=indexing
            tunnel: w576 -> [w588]
            tunnel: w575 -> [w585]
            tunnel: w574 -> [w580]
            tunnel: w573 -> [w579]
            n324 = Unbundle By Name(w587) -> ("Stimulus Data"=w586:dbl[], "Response Data"=w589:dbl[])
            n325 = Bundle(w588, "Stimulus Data"=w586) -> (w582:cluster{dbl[], "Stimulus Data":dbl[]})  [unwired: 1 in]
            n326 = Bundle(w588, "Response Data"=w589) -> (w581:cluster{dbl[], "Response Data":dbl[]})  [unwired: 1 in]
            n327 = call "XY Graph - Append Plot.vi"("Style"=w580, "Data"=w581, "XYGraph Refnum in"=w585) -> ("error out"=w583:errorcluster, "XYGraph Refnum out"=w584:refnum<vi>)  [unwired: 7 in]
            n328 = call "XY Graph - Append Plot.vi"("error in (no error)"=w583, "Style"=w579, "Data"=w582, "XYGraph Refnum in"=w584) -> ()  [unwired: 6 in, 2 out]
          }
          n329 = in-place-dvr #5(w577) -> ()  [unwired: 2 out]
        }
      }
      frame "Plot Saccade Data" {
        # "Plot saccade data to the graph."
        n330 = Unbundle By Name(w596) -> ("Sample Rate (Hz)"=w595:dbl, "Saccades"=w593:T8[], "Impulse Data"=w594:refnum<data-value>, "Palette.Saccade"=w591:u32, "Palette.Excluded Saccade"=w590:u32)
        n331 = control-ref of="graph"() -> (w592:refnum<vi>)
        n332 = for {
          tunnel: w595 -> [w615]
          tunnel: w593 -> [w603] mode=indexing
          tunnel: w594 -> [w614]
          tunnel: w592 -> [w613]
          tunnel: w591 -> [w601]
          tunnel: w590 -> [w600]
          # "Draw each saccade"
          n333 = Unbundle By Name(w603) -> ("Included?"=w602:bool)
          n334 = Select(t=w601, s=w602, f=w600) -> (s? t:f=w599:u32)
          n335 = Bundle By Name(cluster=T17 {"Plot.Anti-aliased"=FALSE, "Plot.Bar Plot Style"=0, "Plot.Digital Line Style"=0, "Plot.Digital Transition Location"=0, "Plot.Digital Transition Type"=0, "Plot.Fill To"=-1, "Plot.Fill/Point Color"=0, "Plot.Label Format"=0, "Plot.Line Style"=0, "Plot.Line Width"=0, "Plot.Plot Color"=0, "Plot.Plot Interpolation"=2, "Plot.Plot Name"="", "Plot.Point Style"=0, "Plot.Visible"=TRUE} ("Style"), "Plot.Plot Color"=w599) -> (w604:T17)
          n336 = Unbundle By Name(w603) -> ("Start (idx)"=w612:dbl, "End (idx)"=w611:dbl)
          n337 = call "ImpulseData - Get Saccade Trace.vi"("Saccade in"=w603, "Impulse Data"=w614) -> ("Response Data"=w607:dbl[])  [unwired: 4 in, 4 out]
          n338 = call "Build dt Ramp.vi"("Stop idx"=w611, "Start idx (0)"=w612, "Frequency (Hz)"=w615) -> ("Ramp (s)"=w609:dbl[])  [unwired: 7 in, 1 out]
          n339 = Multiply(x=w609, y=1000.0) -> (x*y=w610:dbl[])
          n340 = Bundle(w610, "Response Data"=w607) -> (w606:cluster{dbl[], "Response Data":dbl[]})  [unwired: 1 in]
          n341 = call "XY Graph - Append Plot.vi"("Style"=w604, "Data"=w606, "XYGraph Refnum in"=w613) -> ()  [unwired: 7 in, 2 out]
        }
      }
      frame "Fill Saccade MCLB" {
        # "ref obtained again in case N = 0"
        # "Put saccade info in the Saccade MCLB"
        n342 = control-ref of="mclb_saccades"() -> (w617:refnum<vi>)
        n343 = Unbundle By Name(w620) -> ("Saccades"=w619:T8[])
        n344 = for {
          tunnel: w619 -> [w644] mode=indexing
          tunnel: [w627] -> w618 mode=indexing
          tunnel: w617 -> [w632]
          i -> [w633]
          w638 = i16 2  # precision
          # "For each saccade -> Build info string array and colorise rows."
          n345 = Unbundle By Name(w644) -> ("Impulse"=w624:i32, "Sequence #"=w625:dbl, "Onset (ms)"=w626:dbl, "Duration (ms)"=w643:dbl, "Vel (°/s)"=w642:dbl, "Amplitude (°)"=w641:dbl, "Gain"=w640:dbl, "Included?"=w637:bool)
          n346 = Build Array(w624, w625) -> (w623:dbl[])
          n347 = Build Array(w626, w643, w642, w641, w640) -> (w639:dbl[])
          n348 = Number To Decimal String(number=w623) -> (decimal integer string=w628:string[])  [unwired: 1 in]
          n349 = Number To Fractional String(number=w639, precision (6)=w638) -> (F-format string=w629:string[])  [unwired: 2 in]
          n350 = Select(t=u32 0 ("Active Cell:Cell Font:Color"), s=w637, f=u32 13816530 ("Active Cell:Cell Font:Color")) -> (s? t:f=w630:u32)
          n351 = Build Array (concatenate)(w628, w629) -> (w627:string[])
          n352 = Bundle(w633, -2) -> (w631:cluster{i32, i32})  [unwired: 1 in]
          n353 = property class="MCListbox (strict)"(reference=w632, "ActiveCell"=w631, "CellFontColor"=w630) -> ()  [unwired: 1 in, 2 out]
        }
        n354 = control-ref of="mclb_saccades"() -> (w616:refnum<vi>)
        n355 = property class="MCListbox (strict)"(reference=w616, "ItemNames"=w618) -> ()  [unwired: 1 in, 2 out]
      }
      frame "Fill Summary Stats" {
        w659 = i16 2  # precision
        # "Put summary info in the summary MCLB"
        n356 = Unbundle By Name(w658) -> ("Summary.Num Impulses"=w652:dbl, "Summary.Num Saccades"=w651:dbl, "Summary.Onset (ms)"=w657:dbl, "Summary.Duration (ms)"=w656:dbl, "Summary.Vel (°/s)"=w654:dbl, "Summary.Amplitude (°)"=w653:dbl, "Summary.Gain"=w655:dbl)
        n357 = Build Array(w657, w656, w654, w653, w655) -> (w650:dbl[])
        n358 = Build Array(w652, w651) -> (w649:dbl[])
        n359 = Number To Fractional String(number=w650, precision (6)=w659) -> (F-format string=w647:string[])  [unwired: 2 in]
        n360 = Number To Decimal String(number=w649) -> (decimal integer string=w648:string[])  [unwired: 1 in]
        n361 = Build Array (concatenate)(w648, w647) -> (w646:string[])
        n362 = Build Array(w646) -> (w645:string[][])
        n363 = property on="mclb_summary" class="MCListbox (strict)"("ItemNames"=w645) -> ()  [unwired: 2 in, 2 out]
      }
      frame "Halt Panel Updates" {
        # "Defers panel updates preventing GUI updates to front panel controls."
        n364 = control-ref of="This VI"() -> (w664:refnum<vi>)
        n365 = property class="VI"(reference=w664) -> ("Panel"=w663:refnum<vi>)  [unwired: 1 in, 2 out]
        n366 = property class="Pnl"(reference=w663, "Defer Panel Updates"=TRUE) -> ()  [unwired: 1 in, 2 out]
      }
      frame "Resume Panel Updates" {
        # "Resumes panel updates pushing all new GUI info to front panel controls."
        n367 = control-ref of="This VI"() -> (w670:refnum<vi>)
        n368 = property class="VI"(reference=w670) -> ("Panel"=w669:refnum<vi>)  [unwired: 1 in, 2 out]
        n369 = property class="Pnl"(reference=w669, "Defer Panel Updates"=FALSE) -> ()  [unwired: 1 in, 2 out]
      }
      frame "Disable Controls" {
        # "Disable all front panel controls, preventing user interaction."
        n370 = call <userlib>:"MGI Get VI Control Ref[].vi"() -> ("error out"=w675:errorcluster, "Control[i]"=w674:refnum<vi>[])  [unwired: 8 in, 2 out]
        n371 = call <vilib>:"Disable and Grey Group.vi"("error in (no error)"=w675, "Group"=w674) -> ()  [unwired: 8 in, 2 out]